vi "air mod.vi"() -> ()   [LabVIEW 2018]
panel:
  in  "Tab Control":T1(tab)
  in  "Numeric 3":dbl
  in  "Numeric":dbl
  out "fan":dbl(slide) scale=0.0..10.0
  in  "temp-":bool
  in  "temp+":bool
  out "7 2":bool
  out "6 2":bool
  out "5 2":bool
  out "4 2":bool
  out "1 2":bool
  out "7":bool
  out "6":bool
  out "4":bool
  out "3":bool
  out "1":bool
  in  "on/off":bool
  in  "fan-":bool
  in  "fan+":bool
  in  "Numeric 2":dbl
  # "TEMP"
  # "FAN"
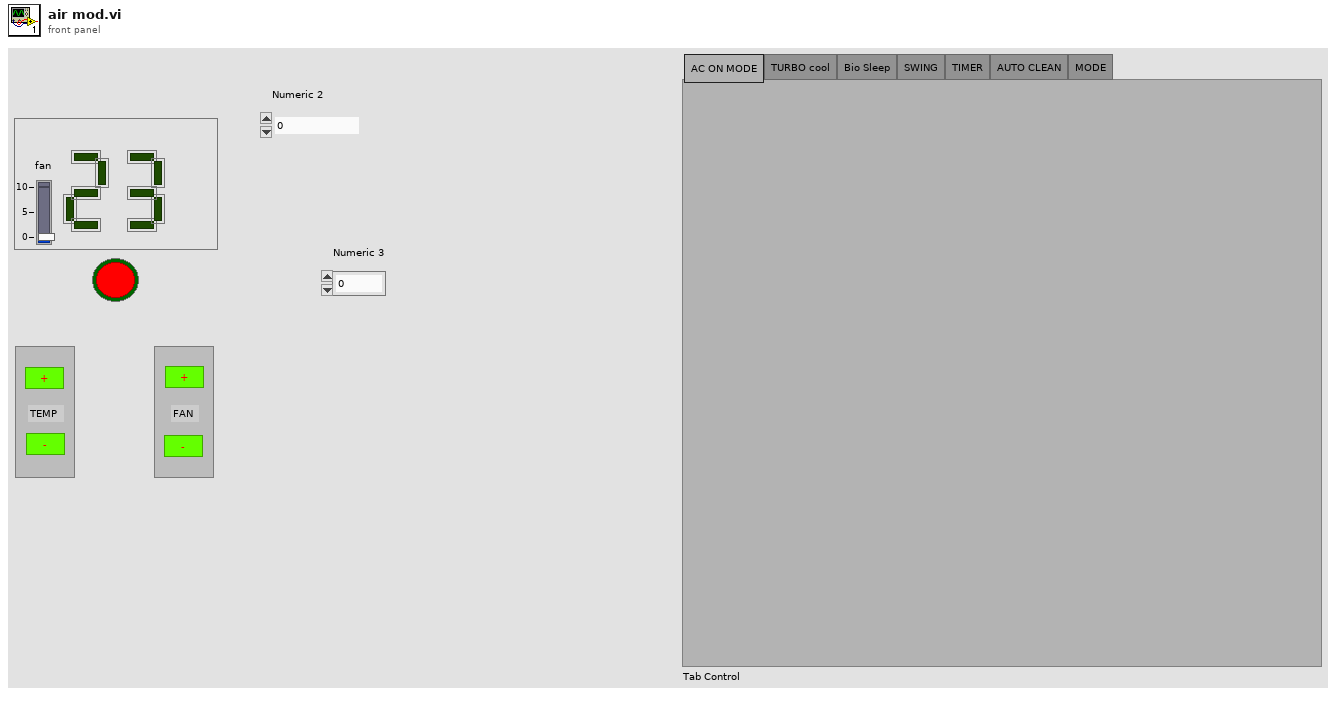
[diagram p1: front panel]
types:
  T1 = enum32{"AC ON MODE", "TURBO cool", "Bio Sleep", "SWING", "TIMER", "AUTO CLEAN", "MODE"}
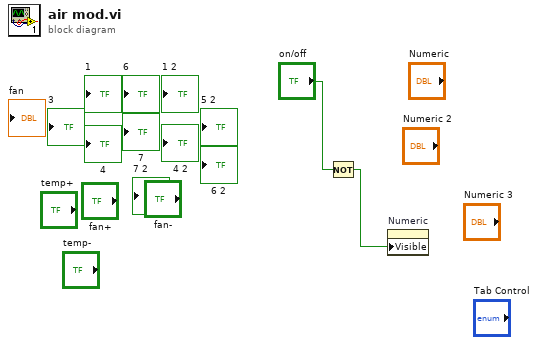
[diagram p0: block diagram]
diagram:
  n1 = Not(x="on/off") -> (.not. x?=w1:bool)
  n2 = property on="Numeric" class="DigNum (strict)"("Visible"=w1) -> ()  [unwired: 2 in, 2 out]
